vi "Move Picture Demo.vi"() -> ()   [LabVIEW 2012, in "Picture Box Tools.lvlib"]
uses:
  Picture Box Tools.lvlib
  <vilib>/picture/picture.llb/imagedata.ctl
  Rectangle Tools/Rect/OffsetRect/OffsetRect by HV and Rect.vi
  Rectangle Tools/Rect/Rect Tools.lvlib
panel:
  in  "Step":i16=5
  in  "Up":bool
  in  "Left":bool
  in  "Right":bool
  in  "Down":bool
  in  "停止按钮":bool
  out "二维图片":picture
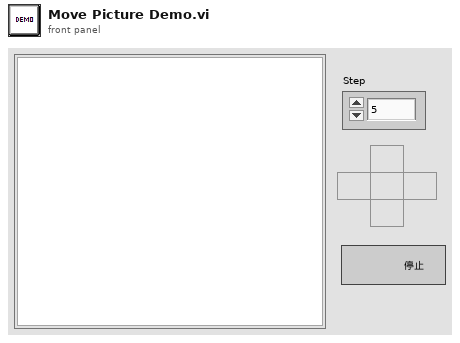
[diagram p1: front panel]
types:
  T1 = typedef "imagedata.ctl" = cluster{"image type":i32, "image depth":i32, "image":u8[], "mask":u8[], "colors":u32[], "Rectangle":cluster{"left":i16, "top":i16, "right":i16, "bottom":i16}}
  T2 = cluster{"left":i16, "top":i16, "right":i16, "bottom":i16}
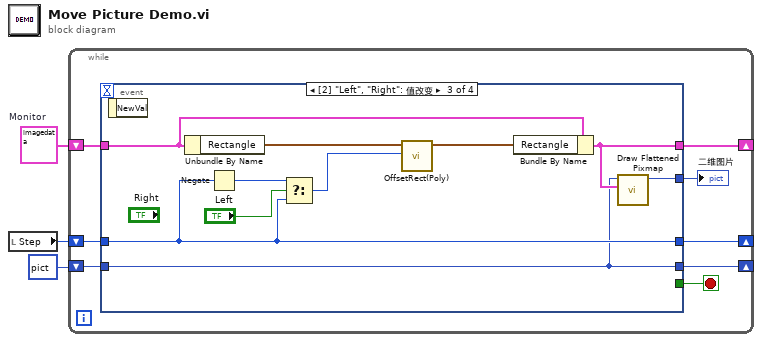
[diagram p0: block diagram]
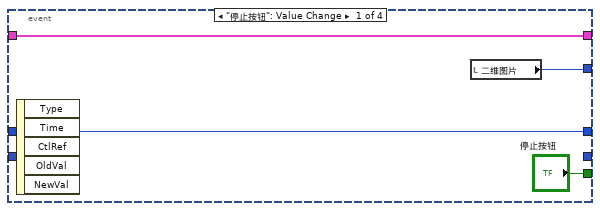
[diagram p2: hidden frame]
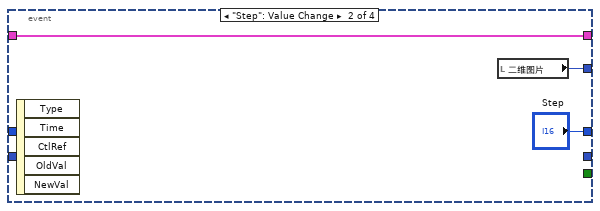
[diagram p3: hidden frame]
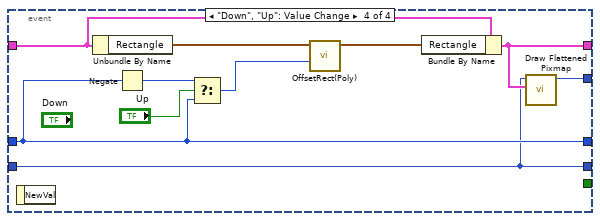
[diagram p4: hidden frame]
diagram:
  w2 = T1 {"image type"=0, "image depth"=24, "image"=[198, 198, 198, 0, 0, 0, 0, 0, 0, 0, 0, 0, 0, 0, 0, 0, 0, 0, 0, 0, 0, 0, 0, 0, 0, 0, 0, 0, 0, 0, 0, 0, 0, 0, 0, 0, 0, 0, 0, 0, 0, 0, 0, 0, 0, 255, 255, 255, 0, 0, 0, 214, 214, 214, 255, 255, 255, 255, 255, 255, 255, 255, 255, 255, 255, 255, 255, 255, 255, 255, 255, 255, 255, 255, 255, 255, 255, 255, 239, 239, 239, 239, 239, 239, 239, 239, 239, 239, 239, 239, 198, 198, 198, 0, 0, 0, 0, 0, 0, 255, 255, 255, 0, 0, 0, 0, 0, 0, 0, 0, 0, 0, 0, 0, 0, 0, 0, 0, 0, 0, 0, 0, 0, 0, 0, 0, 0, 0, 0, 0, 0, 0, 0, 0, 0, 0, 0, 0, 198, 198, 198, 0, 0, 0, 0, 0, 0, 255, 255, 255, 0, 0, 0, 222, 239, 239, 214, 239, 239, 198, 231, 231, 189, 222, 222, 181, 222, 222, 165, 214, 214, 156, 206, 206, 156, 206, 206, 132, 198, 198, 107, 181, 181, 0, 0, 0, 198, 198, 198, 0, 0, 0, 0, 0, 0, 255, 255, 255, 0, 0, 0, 198, 231, 231, 189, 222, 222, 181, 222, 222, 165, 214, 214, 156, 206, 206, 156, 206, 206, 132, 198, 198, 132, 198, 198, 107, 181, 181, 99, 181, 181, 0, 0, 0, 198, 198, 198, 0, 0, 0, 0, 0, 0, 255, 255, 255, 0, 0, 0, 181, 222, 222, 165, 214, 214, 156, 206, 206, 156, 206, 206, 140, 198, 198, 132, 198, 198, 123, 189, 189, 107, 181, 181, 99, 181, 181, 74, 165, 165, 0, 0, 0, 198, 198, 198, 0, 0, 0, 0, 0, 0, 255, 255, 255, 0, 0, 0, 165, 214, 214, 156, 206, 206, 156, 206, 206, 140, 198, 198, 132, 198, 198, 107, 181, 181, 99, 181, 181, 99, 181, 181, 74, 165, 165, 66, 165, 165, 0, 0, 0, 198, 198, 198, 0, 0, 0, 0, 0, 0, 255, 255, 255, 0, 0, 0, 156, 206, 206, 140, 198, 198, 132, 198, 198, 123, 189, 189, 107, 181, 181, 99, 181, 181, 82, 173, 173, 74, 165, 165, 66, 165, 165, 49, 156, 156, 0, 0, 0, 198, 198, 198, 0, 0, 0, 0, 0, 0, 255, 255, 255, 0, 0, 0, 140, 198, 198, 132, 198, 198, 123, 189, 189, 107, 181, 181, 99, 181, 181, 82, 173, 173, 74, 165, 165, 66, 165, 165, 41, 148, 148, 41, 148, 148, 0, 0, 0, 198, 198, 198, 0, 0, 0, 0, 0, 0, 255, 255, 255, 0, 0, 0, 132, 198, 198, 123, 189, 189, 107, 181, 181, 99, 181, 181, 82, 173, 173, 74, 165, 165, 66, 165, 165, 41, 148, 148, 24, 140, 140, 16, 140, 140, 0, 0, 0, 198, 198, 198, 0, 0, 0, 0, 0, 0, 255, 255, 255, 0, 0, 0, 123, 189, 189, 107, 181, 181, 99, 181, 181, 82, 173, 173, 74, 165, 165, 66, 165, 165, 49, 156, 156, 41, 148, 148, 24, 140, 140, 16, 140, 140, 0, 0, 0, 198, 198, 198, 0, 0, 0, 0, 0, 0, 255, 255, 255, 0, 0, 0, 0, 0, 0, 0, 0, 0, 0, 0, 0, 0, 0, 0, 0, 0, 0, 0, 0, 0, 0, 0, 0, 0, 0, 0, 0, 0, 0, 0, 0, 0, 0, 0, 0, 198, 198, 198, 0, 0, 0, 0, 0, 0, 198, 198, 198, 198, 198, 198, 198, 198, 198, 198, 198, 198, 198, 198, 198, 198, 198, 198, 198, 198, 198, 198, 198, 198, 198, 198, 198, 198, 198, 198, 198, 198, 198, 198, 198, 198, 198, 198, 198, 198, 198, 198, 0, 0, 0, 255, 255, 255, 0, 0, 0, 0, 0, 0, 0, 0, 0, 0, 0, 0, 0, 0, 0, 0, 0, 0, 0, 0, 0, 0, 0, 0, 0, 0, 0, 0, 0, 0, 0, 0, 0, 0, 0, 0, 0, 0, 0, 0, 0, 0, 255, 255, 255], "mask"=[], "colors"=[], "Rectangle"={"left"=0, "top"=0, "right"=16, "bottom"=14}}  # Monitor
  n1 = local read "Step"() -> (w3:i16)
  n2 = while {
    shift-right: [w9] -> _
    shift-left: w3 -> [w10]
    shift-right: [w8] -> _
    shift-left: w2 -> [w7]
    shift-right: [w4] -> _
    shift-left: picture bytes[3145758] ("二维图片") -> [w5]
    stop <- w11 stop-if-true
    n3 = event shown="[2] \"Left\", \"Right\": 值改变" {
      selector: _ -> [_ _ _ _]
      dyn-events: _ -> [_ _ _ _]
      timeout: _ -> [_ _ _ _]
      tunnel: ["停止按钮" _ _ _] -> w11
      tunnel: w10 -> [w14 _ w24 w32]
      tunnel: [w14 "Step" w24 w32] -> w9
      tunnel: w7 -> [w13 w17 w22 w35]
      tunnel: [w13 w17 w27 w34] -> w8
      tunnel: [w12 w16 w20 w30] -> w6
      tunnel: w5 -> [_ _ w19 w29]
      tunnel: [_ _ w19 w29] -> w4
      event "停止按钮": Value Change {
        n4 = event-data() -> ()  [unwired: 1 in, 5 out]
        n5 = local read "二维图片"() -> (w12:picture)
      }
      event "Step": Value Change {
        n6 = event-data() -> ()  [unwired: 1 in, 5 out]
        n7 = local read "二维图片"() -> (w16:picture)
      }
      event "Left", "Right": Value Change {
        n8 = event-data() -> ()  [unwired: 1 in, 1 out]
        n9 = Unbundle By Name(w22) -> ("Rectangle"=w21:T2)
        n10 = Negate(x=w24) -> (-x=w25:i16)
        n11 = Select(t=w25, s="Left", f=w24) -> (s? t:f=w23:i16)
        n12 = call-poly "OffsetRect(Poly).vi"("h"=w23, "rect"=w21) -> ("offset rect"=w28:T2)  [unwired: 8 in, 1 out]
        n13 = Bundle By Name(cluster=w22, "Rectangle"=w28) -> (w27:T1)
        n14 = call <vilib>:"Draw Flattened Pixmap.vi"("image data"=w27, "picture"=w19) -> ("new picture"=w20:picture)  [unwired: 7 in]
      }
      event "Down", "Up": Value Change {
        n15 = event-data() -> ()  [unwired: 1 in, 1 out]
        n16 = Unbundle By Name(w35) -> ("Rectangle"=w36:T2)
        n17 = Negate(x=w32) -> (-x=w37:i16)
        n18 = Select(t=w37, s="Up", f=w32) -> (s? t:f=w31:i16)
        n19 = call-poly "OffsetRect(Poly).vi"("v"=w31, "rect"=w36) -> ("offset rect"=w38:T2)  [unwired: 8 in, 1 out]
        n20 = Bundle By Name(cluster=w35, "Rectangle"=w38) -> (w34:T1)
        n21 = call <vilib>:"Draw Flattened Pixmap.vi"("image data"=w34, "picture"=w29) -> ("new picture"=w30:picture)  [unwired: 7 in]
      }
    }
    "二维图片" <- w6
  }
